vi "ZMQ PAIR sender example.vi"() -> ()   [LabVIEW 2018]
uses:
  <vilib>/addons/zeromq/socket_type.ctl
  <vilib>/addons/zeromq/zeromq.lvlib
  <vilib>/addons/zeromq/zmq_context.lvclass
  <vilib>/addons/zeromq/zmq_socket.lvclass
panel:
  out "string flatten time":u32
  in  "Stop":bool
  out "message":string[](array[string])
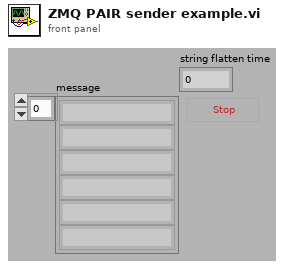
[diagram p1: front panel]
types:
  T1 = typedef "zeromq.lvlib/socket_type.ctl" = enum8{"ZMQ_PAIR", "ZMQ_PUB", "ZMQ_SUB", "ZMQ_REQ", "ZMQ_REP", "ZMQ_DEALER", "ZMQ_ROUTER", "ZMQ_PULL", "ZMQ_PUSH", "ZMQ_XPUB", "ZMQ_XSUB"}
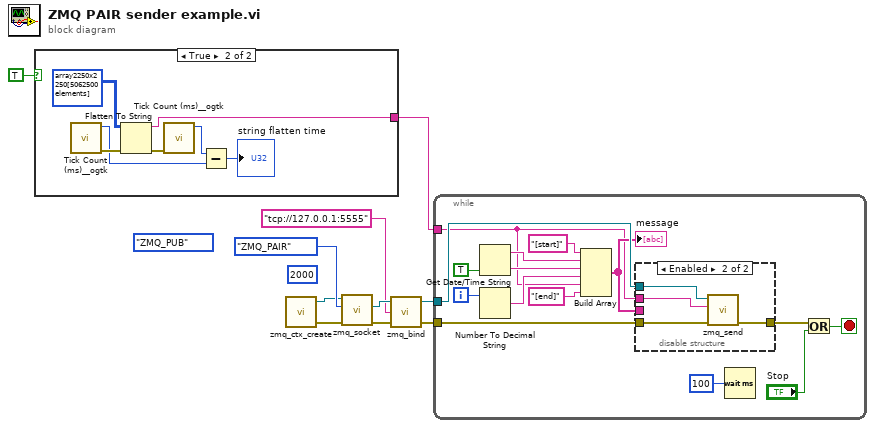
[diagram p0: block diagram]
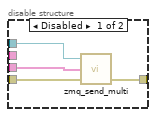
[diagram p3: hidden frame]
diagram:
  (unwired) socket_type."ZMQ_PUB" ("socket type")
  (unwired) 2000 ("linger (ms)")
  n1 = case shown="True" TRUE {
    tunnel: [_ w16] -> w2
    frame False {
    }
    frame True {
      n2 = call <userlib>:"Tick Count (ms)__ogtk.vi"() -> ("error out"=w15:errorcluster, "millisecond timer value"=w12:u32)  [unwired: 10 in]
      n3 = Flatten To String(anything=u16[][] array2250x2250[5062500 elements] ("Array"), error in (no error)=w15) -> (data string=w16:string, error out=w14:errorcluster)  [unwired: 2 in, 1 out]
      n4 = call <userlib>:"Tick Count (ms)__ogtk.vi"("error in (no error)"=w14) -> ("millisecond timer value"=w13:u32)  [unwired: 9 in, 1 out]
      n5 = Subtract(x=w13, y=w12) -> (x-y=→"string flatten time":u32)
    }
  }
  n6 = call <vilib>:"zmq_ctx_create.vi"() -> ("error out"=w8:errorcluster, "context out"=w5:refnum<class "zmq_context.lvclass">)  [unwired: 4 in]
  n7 = call <vilib>:"zmq_socket.vi"("error in"=w8, "socket type"=socket_type."ZMQ_PAIR", "context in"=w5) -> ("error out"=w7:errorcluster, "socket out"=w4:refnum<class "zmq_socket.lvclass">)  [unwired: 2 in, 1 out]
  n8 = call <vilib>:"zmq_bind.vi"("error in"=w7, "endpoint"="tcp://127.0.0.1:5555", "socket in"=w4) -> ("error out"=w6:errorcluster, "socket out"=w10:refnum<class "zmq_socket.lvclass">)  [unwired: 1 in]
  n9 = while {
    tunnel: w10 -> [w31]
    tunnel: w6 -> [w30]
    tunnel: w2 -> [w18]
    i -> [w24]
    stop <- w21 stop-if-true
    n10 = Get Date/Time String(want seconds? (F)=TRUE) -> (date string=w29:string, time string=w28:string)  [unwired: 2 in]
    n11 = Number To Decimal String(number=w24) -> (decimal integer string=w25:string)  [unwired: 1 in]
    n12 = Build Array("[start]" ("element"), w29, w28, w25, w18, "[end]" ("element")) -> (w19:string[])
    "message" <- w19
    n13 = disable-structure shown="Enabled" {
      disable-tunnel: w31 -> [w36 w40]
      disable-tunnel: w30 -> [w35 w38]
      disable-tunnel: [w34 w37] -> w22
      disable-tunnel: w19 -> [w33 _]
      disable-tunnel: w18 -> [_ w39]
      frame Disabled {
        n14 = call <vilib>:"zmq_send_multi.vi"("error in"=w35, "parts"=w33, "socket in"=w36) -> ("error out"=w34:errorcluster)  [unwired: 1 in, 1 out]
      }
      frame Enabled {
        n15 = call <vilib>:"zmq_send.vi"("error in"=w38, "data"=w39, "socket in"=w40) -> ("error out"=w37:errorcluster)  [unwired: 4 in, 1 out]
      }
    }
    n16 = Wait (ms)(milliseconds to wait=u32 100) -> ()  [unwired: 1 out]
    n17 = Or(x=w22, y="Stop") -> (x .or. y?=w21:bool)
  }
